vi "Dresden R2R Sputter 03.02.2018 IY24.vi"() -> ()   [LabVIEW 2009] (continued)
                                }
                                }
                                }
                                frame #1 {
                                n15635 = local read "Semi"() -> (w27616)
                                n15636 = case shown="False" w27616 {
                                frame #0 {
                                n15637 = local write "Ch1_PV18"(T/1 ("P03")) -> ()
                                n15638 = Wait Until Next ms Multiple(millisecond multiple=i32? 1000) -> ()  [unwired: 1 out]
                                }
                                frame #1 {
                                }
                                }
                                }
                                }
                              }
                              frame #1 {
                              }
                            }
                          }
                          frame #13 {
                            # "START TP"
                            n15639 = local read "Semi"() -> (w27619)
                            n15640 = case shown="False" w27619 {
                              frame #0 {
                                n15641 = stacked-sequence {
                                frame #0 {
                                n15642 = local read "Semi"() -> (w27620)
                                n15643 = case shown="False" w27620 {
                                frame #0 {
                                n15644 = stacked-sequence {
                                frame #0 {
                                n15645 = local read "Semi"() -> (w27621)
                                n15646 = case shown="False" w27621 {
                                frame #0 {
                                n15647 = local write "Tp1_auto_start"(T/1 ("Tp1_auto_start")) -> ()
                                }
                                frame #1 {
                                }
                                }
                                }
                                frame #1 {
                                n15648 = local read "Semi"() -> (w27623)
                                n15649 = case shown="False" w27623 {
                                frame #0 {
                                n15650 = Wait (ms)(milliseconds to wait=i32? 1000) -> ()  [unwired: 1 out]
                                }
                                frame #1 {
                                }
                                }
                                }
                                frame #2 {
                                n15651 = local read "Semi"() -> (w27625)
                                n15652 = case shown="False" w27625 {
                                frame #0 {
                                n15653 = while {
                                i -> [w27631]
                                stop <- w27627 stop-if-true
                                n15654 = local read "TP1_working"() -> (w27629)
                                n15655 = Greater?(x=w27631, y=i32? 120) -> (0:w27630)
                                n15656 = local read "Semi"() -> (w27628)
                                n15657 = Compound Arithmetic op=OR(w27628, w27629, w27630) -> (w27627)
                                n15658 = Wait (ms)(milliseconds to wait=i32? 500) -> ()  [unwired: 1 out]
                                }
                                }
                                frame #1 {
                                }
                                }
                                }
                                frame #3 {
                                n15659 = local read "Semi"() -> (w27633)
                                n15660 = case shown="False" w27633 {
                                frame #0 {
                                n15661 = local read "TP1_working"() -> (w27634)
                                n15662 = case shown="False" w27634 {
                                frame #0 {
                                n15663 = local write "Tp1_auto_start"(T/1 ("Pc_bv1_auto_open")) -> ()
                                }
                                frame #1 {
                                }
                                }
                                }
                                frame #1 {
                                }
                                }
                                }
                                frame #4 {
                                n15664 = local read "Semi"() -> (w27636)
                                n15665 = case shown="False" w27636 {
                                frame #0 {
                                n15666 = local read "TP1_working"() -> (w27637)
                                n15667 = case shown="False" w27637 {
                                frame #0 {
                                n15668 = Wait (ms)(milliseconds to wait=i32? 1000) -> ()  [unwired: 1 out]
                                }
                                frame #1 {
                                }
                                }
                                }
                                frame #1 {
                                }
                                }
                                }
                                frame #5 {
                                n15669 = local read "Semi"() -> (w27639)
                                n15670 = case shown="False" w27639 {
                                frame #0 {
                                n15671 = while {
                                i -> [w27645]
                                stop <- w27641 stop-if-true
                                n15672 = local read "TP1_working"() -> (w27643)
                                n15673 = Greater?(x=w27645, y=i32? 120) -> (0:w27644)
                                n15674 = local read "Semi"() -> (w27642)
                                n15675 = Compound Arithmetic op=OR(w27642, w27643, w27644) -> (w27641)
                                n15676 = Wait (ms)(milliseconds to wait=i32? 500) -> ()  [unwired: 1 out]
                                }
                                }
                                frame #1 {
                                }
                                }
                                }
                                frame #6 {
                                n15677 = local read "Semi"() -> (w27647)
                                n15678 = case shown="False" w27647 {
                                frame #0 {
                                n15679 = local read "TP1_working"() -> (w27648)
                                n15680 = case shown="False" w27648 {
                                frame #0 {
                                n15681 = local write "Error Message"("Start up process  cancelled\nbecause  TP not started.\nPlease check TP1 connections." ("Error Message")) -> ()
                                n15682 = Wait (ms)(milliseconds to wait=i32? 1000) -> ()  [unwired: 1 out]
                                }
                                frame #1 {
                                }
                                }
                                }
                                frame #1 {
                                }
                                }
                                }
                                }
                                }
                                frame #1 {
                                }
                                }
                                }
                                frame #1 {
                                n15683 = local read "Semi"() -> (w27651)
                                n15684 = case shown="False" w27651 {
                                frame #0 {
                                n15685 = local write "Ch1_PV19"(T/1 ("P03")) -> ()
                                n15686 = Wait Until Next ms Multiple(millisecond multiple=i32? 1000) -> ()  [unwired: 1 out]
                                }
                                frame #1 {
                                }
                                }
                                }
                                }
                              }
                              frame #1 {
                              }
                            }
                          }
                        }
                      }
                      frame #1 {
                      }
                    }
                  }
                  frame #1 {
                    # "PUMPING CH1 HIGHER THAN 0.9 TORR"
                    n15687 = local read "Semi"() -> (w27654)
                    n15688 = case shown="False" w27654 {
                      frame #0 {
                        n15689 = stacked-sequence {
                          frame #0 {
                            # "STOP TP"
                            n15690 = local read "Semi"() -> (w27655)
                            n15691 = case shown="False" w27655 {
                              frame #0 {
                                n15692 = stacked-sequence {
                                frame #0 {
                                n15693 = local read "Semi"() -> (w27656)
                                n15694 = case shown="False" w27656 {
                                frame #0 {
                                n15695 = stacked-sequence {
                                frame #0 {
                                n15696 = local read "Semi"() -> (w27657)
                                n15697 = case shown="False" w27657 {
                                frame #0 {
                                n15698 = local write "Tp1_auto_stop"(T/1 ("Tp1_auto_start")) -> ()
                                }
                                frame #1 {
                                }
                                }
                                }
                                frame #1 {
                                n15699 = local read "Semi"() -> (w27659)
                                n15700 = case shown="False" w27659 {
                                frame #0 {
                                n15701 = Wait (ms)(milliseconds to wait=i32? 1000) -> ()  [unwired: 1 out]
                                }
                                frame #1 {
                                }
                                }
                                }
                                frame #2 {
                                n15702 = local read "Semi"() -> (w27661)
                                n15703 = case shown="False" w27661 {
                                frame #0 {
                                n15704 = while {
                                i -> [w27667]
                                stop <- w27663 stop-if-true
                                n15705 = local read "Tp1_stopped"() -> (w27665)
                                n15706 = Greater?(x=w27667, y=i32? 120) -> (0:w27666)
                                n15707 = local read "Semi"() -> (w27664)
                                n15708 = Compound Arithmetic op=OR(w27664, w27665, w27666) -> (w27663)
                                n15709 = Wait (ms)(milliseconds to wait=i32? 500) -> ()  [unwired: 1 out]
                                }
                                }
                                frame #1 {
                                }
                                }
                                }
                                frame #3 {
                                n15710 = local read "Semi"() -> (w27669)
                                n15711 = case shown="False" w27669 {
                                frame #0 {
                                n15712 = local read "Tp1_stopped"() -> (w27670)
                                n15713 = case shown="False" w27670 {
                                frame #0 {
                                n15714 = local write "Tp1_auto_stop"(T/1 ("Pc_bv1_auto_open")) -> ()
                                }
                                frame #1 {
                                }
                                }
                                }
                                frame #1 {
                                }
                                }
                                }
                                frame #4 {
                                n15715 = local read "Semi"() -> (w27672)
                                n15716 = case shown="False" w27672 {
                                frame #0 {
                                n15717 = local read "Tp1_stopped"() -> (w27673)
                                n15718 = case shown="False" w27673 {
                                frame #0 {
                                n15719 = Wait (ms)(milliseconds to wait=i32? 1000) -> ()  [unwired: 1 out]
                                }
                                frame #1 {
                                }
                                }
                                }
                                frame #1 {
                                }
                                }
                                }
                                frame #5 {
                                n15720 = local read "Semi"() -> (w27675)
                                n15721 = case shown="False" w27675 {
                                frame #0 {
                                n15722 = while {
                                i -> [w27681]
                                stop <- w27677 stop-if-true
                                n15723 = local read "Tp1_stopped"() -> (w27679)
                                n15724 = Greater?(x=w27681, y=i32? 120) -> (0:w27680)
                                n15725 = local read "Semi"() -> (w27678)
                                n15726 = Compound Arithmetic op=OR(w27678, w27679, w27680) -> (w27677)
                                n15727 = Wait (ms)(milliseconds to wait=i32? 500) -> ()  [unwired: 1 out]
                                }
                                }
                                frame #1 {
                                }
                                }
                                }
                                frame #6 {
                                n15728 = local read "Semi"() -> (w27683)
                                n15729 = case shown="False" w27683 {
                                frame #0 {
                                n15730 = local read "Tp1_stopped"() -> (w27684)
                                n15731 = case shown="False" w27684 {
                                frame #0 {
                                n15732 = local write "Error Message"("Start up process  cancelled\nbecause  TP not stopped.\nPlease check TP1 connections." ("Error Message")) -> ()
                                n15733 = Wait (ms)(milliseconds to wait=i32? 1000) -> ()  [unwired: 1 out]
                                }
                                frame #1 {
                                }
                                }
                                }
                                frame #1 {
                                }
                                }
                                }
                                }
                                }
                                frame #1 {
                                }
                                }
                                }
                                frame #1 {
                                n15734 = local read "Semi"() -> (w27687)
                                n15735 = case shown="False" w27687 {
                                frame #0 {
                                n15736 = local write "Ch1_PA6"(T/1 ("PA2")) -> ()
                                n15737 = Wait Until Next ms Multiple(millisecond multiple=i32? 1000) -> ()  [unwired: 1 out]
                                }
                                frame #1 {
                                }
                                }
                                }
                                }
                              }
                              frame #1 {
                              }
                            }
                          }
                          frame #1 {
                            # "CLOSE CH1-CC"
                            n15738 = local read "Semi"() -> (w27690)
                            n15739 = case shown="False" w27690 {
                              frame #0 {
                                n15740 = stacked-sequence {
                                frame #0 {
                                n15741 = local read "Semi"() -> (w27691)
                                n15742 = case shown="False" w27691 {
                                frame #0 {
                                n15743 = while {
                                i -> [w27698]
                                stop <- w27692 stop-if-true
                                n15744 = Greater?(x=w27698, y=i32? 50) -> (0:w27696)
                                n15745 = case shown="True" w27696 {
                                frame #0 {
                                }
                                frame #1 {
                                n15746 = local write "Semi"(T/1 ("Semi")) -> ()
                                n15747 = local write "Error Message"("Start up process  cancelled\nbecause  CH1-CC not closed.\nPlease check  CH1-CC connections." ("Error Message")) -> ()
                                }
                                }
                                n15748 = local read "Ch1_Cc_on_off_di"() -> (w27695)
                                n15749 = case shown="True" w27695 {
                                tunnel: [T/1 i16? 0] -> w27694
                                frame #0 {
                                }
                                frame #1 {
                                n15750 = Wait Until Next ms Multiple(millisecond multiple=i32? 200) -> ()  [unwired: 1 out]
                                n15751 = local write "Ch1_Cc_on_off_do"(i16? 0 ("Ch1_Tp_bv_do")) -> ()
                                }
                                }
                                n15752 = local read "Semi"() -> (w27693)
                                n15753 = Or(x=w27694, y=w27693) -> (x .or. y?=w27692)
                                }
                                }
                                frame #1 {
                                }
                                }
                                }
                                frame #1 {
                                n15754 = local read "Semi"() -> (w27705)
                                n15755 = case shown="False" w27705 {
                                frame #0 {
                                n15756 = local write "Ch1_PA7"(T/1 ("PA3")) -> ()
                                n15757 = Wait Until Next ms Multiple(millisecond multiple=i32? 1000) -> ()  [unwired: 1 out]
                                }
                                frame #1 {
                                }
                                }
                                }
                                }
                              }
                              frame #1 {
                              }
                            }
                          }
                          frame #2 {
                            # "CLOSE BG-BV"
                            n15758 = local read "Semi"() -> (w27708)
                            n15759 = case shown="False" w27708 {
                              frame #0 {
                                n15760 = stacked-sequence {
                                frame #0 {
                                n15761 = local read "Semi"() -> (w27709)
                                n15762 = case shown="False" w27709 {
                                frame #0 {
                                n15763 = while {
                                i -> [w27716]
                                stop <- w27710 stop-if-true
                                n15764 = Greater?(x=w27716, y=i32? 50) -> (0:w27714)
                                n15765 = case shown="True" w27714 {
                                frame #0 {
                                }
                                frame #1 {
                                n15766 = local write "Semi"(T/1 ("Semi")) -> ()
                                n15767 = local write "Error Message"("Start up process  cancelled\nbecause  BG-BV not closed.\nPlease check  BG-BV1 connections." ("Error Message")) -> ()
                                }
                                }
                                n15768 = local read "Ch1_Bg_bv_di"() -> (w27713)
                                n15769 = case shown="True" w27713 {
                                tunnel: [T/1 i16? 0] -> w27712
                                frame #0 {
                                }
                                frame #1 {
                                n15770 = Wait Until Next ms Multiple(millisecond multiple=i32? 200) -> ()  [unwired: 1 out]
                                n15771 = local write "Ch1_Bg_bv_do"(i16? 0 ("Ch1_Tp_bv_do")) -> ()
                                }
                                }
                                n15772 = local read "Semi"() -> (w27711)
                                n15773 = Or(x=w27712, y=w27711) -> (x .or. y?=w27710)
                                }
                                }
                                frame #1 {
                                }
                                }
                                }
                                frame #1 {
                                n15774 = local read "Semi"() -> (w27723)
                                n15775 = case shown="False" w27723 {
                                frame #0 {
                                n15776 = local write "Ch1_PA8"(T/1 ("PA3")) -> ()
                                n15777 = Wait Until Next ms Multiple(millisecond multiple=i32? 1000) -> ()  [unwired: 1 out]
                                }
                                frame #1 {
                                }
                                }
                                }
                                }
                              }
                              frame #1 {
                              }
                            }
                          }
                          frame #3 {
                            # "CLOSE TP-BV"
                            n15778 = local read "Semi"() -> (w27726)
                            n15779 = case shown="False" w27726 {
                              frame #0 {
                                n15780 = stacked-sequence {
                                frame #0 {
                                n15781 = local read "Semi"() -> (w27727)
                                n15782 = case shown="False" w27727 {
                                frame #0 {
                                n15783 = while {
                                i -> [w27734]
                                stop <- w27728 stop-if-true
                                n15784 = Greater?(x=w27734, y=i32? 50) -> (0:w27732)
                                n15785 = case shown="True" w27732 {
                                frame #0 {
                                }
                                frame #1 {
                                n15786 = local write "Semi"(T/1 ("Semi")) -> ()
                                n15787 = local write "Error Message"("Start up process  cancelled\nbecause  TP-BV not closed.\nPlease check  TP1-BV connections." ("Error Message")) -> ()
                                }
                                }
                                n15788 = local read "Ch1_Tp_bv_di"() -> (w27731)
                                n15789 = case shown="True" w27731 {
                                tunnel: [T/1 i16? 0] -> w27730
                                frame #0 {
                                }
                                frame #1 {
                                n15790 = Wait Until Next ms Multiple(millisecond multiple=i32? 200) -> ()  [unwired: 1 out]
                                n15791 = local write "Ch1_Tp_bv_do"(i16? 0 ("Ch1_Tp_bv_do")) -> ()
                                }
                                }
                                n15792 = local read "Semi"() -> (w27729)
                                n15793 = Or(x=w27730, y=w27729) -> (x .or. y?=w27728)
                                }
                                }
                                frame #1 {
                                }
                                }
                                }
                                frame #1 {
                                n15794 = local read "Semi"() -> (w27741)
                                n15795 = case shown="False" w27741 {
                                frame #0 {
                                n15796 = local write "Ch1_PA9"(T/1 ("PA5")) -> ()
                                n15797 = Wait Until Next ms Multiple(millisecond multiple=i32? 1000) -> ()  [unwired: 1 out]
                                }
                                frame #1 {
                                }
                                }
                                }
                                }
                              }
                              frame #1 {
                              }
                            }
                          }
                          frame #4 {
                            # "False PL1-ATM"
                            n15798 = local read "Semi"() -> (w27744)
                            n15799 = case shown="False" w27744 {
                              frame #0 {
                                n15800 = stacked-sequence {
                                frame #0 {
                                n15801 = local read "Semi"() -> (w27745)
                                n15802 = case shown="False" w27745 {
                                frame #0 {
                                n15803 = local write "Ch1_Pl_atm_do"(i16? 0 ("Ch1_Pl_atm_do")) -> ()
                                }
                                frame #1 {
                                }
                                }
                                }
                                frame #1 {
                                n15804 = local read "Semi"() -> (w27747)
                                n15805 = case shown="False" w27747 {
                                frame #0 {
                                n15806 = local write "Ch1_PA10"(T/1 ("PA3")) -> ()
                                n15807 = Wait Until Next ms Multiple(millisecond multiple=i32? 1000) -> ()  [unwired: 1 out]
                                }
                                frame #1 {
                                }
                                }
                                }
                                }
                              }
                              frame #1 {
                              }
                            }
                          }
                          frame #5 {
                            # "STOP MP"
                            n15808 = local read "Semi"() -> (w27750)
                            n15809 = case shown="False" w27750 {
                              frame #0 {
                                n15810 = stacked-sequence {
                                frame #0 {
                                n15811 = local read "Semi"() -> (w27751)
                                n15812 = case shown="False" w27751 {
                                frame #0 {
                                n15813 = while {
                                i -> [w27758]
                                stop <- w27752 stop-if-true
                                n15814 = Greater?(x=w27758, y=i32? 50) -> (0:w27756)
                                n15815 = case shown="True" w27756 {
                                frame #0 {
                                }
                                frame #1 {
                                n15816 = local write "Semi"(T/1 ("Semi")) -> ()
                                n15817 = local write "Error Message"("Start up process  cancelled\nbecause MP1 not stopped.\nPlease check MP1 connections." ("Error Message")) -> ()
                                }
                                }
                                n15818 = local read "Ch1_Mp_di"() -> (w27755)
                                n15819 = case shown="True" w27755 {
                                tunnel: [T/1 i16? 0] -> w27754
                                frame #0 {
                                }
                                frame #1 {
                                n15820 = Wait Until Next ms Multiple(millisecond multiple=i32? 200) -> ()  [unwired: 1 out]
                                n15821 = local write "Ch1_Mp_do"(i16? 0 ("Ch1_Tp_bv_do")) -> ()
                                }
                                }
                                n15822 = local read "Semi"() -> (w27753)
                                n15823 = Or(x=w27754, y=w27753) -> (x .or. y?=w27752)
                                }
                                }
                                frame #1 {
                                }
                                }
                                }
                                frame #1 {
                                n15824 = local read "Semi"() -> (w27765)
                                n15825 = case shown="False" w27765 {
                                frame #0 {
                                n15826 = local write "Ch1_PA11"(T/1 ("PA3")) -> ()
                                n15827 = Wait Until Next ms Multiple(millisecond multiple=i32? 1000) -> ()  [unwired: 1 out]
                                }
                                frame #1 {
                                }
                                }
                                }
                                }
                              }
                              frame #1 {
                              }
                            }
                          }
                          frame #6 {
                            # "OPEN PL-VBV1"
                            n15828 = local read "Semi"() -> (w27768)
                            n15829 = case shown="False" w27768 {
                              frame #0 {
                                n15830 = stacked-sequence {
                                frame #0 {
                                n15831 = local read "Semi"() -> (w27769)
                                n15832 = case shown="False" w27769 {
                                frame #0 {
                                n15833 = while {
                                i -> [w27776]
                                stop <- w27771 stop-if-true
                                n15834 = Greater?(x=w27776, y=i32? 50) -> (0:w27774)
                                n15835 = case shown="True" w27774 {
                                frame #0 {
                                }
                                frame #1 {
                                n15836 = local write "Semi"(T/1 ("Semi")) -> ()
                                n15837 = local write "Error Message"("Start up process  cancelled\nbecause  PL-VBV not opened.\nPlease check PL-VBV1 connections." ("Error Message")) -> ()
                                }
                                }
                                n15838 = local read "Ch1_Pl_atm_di"() -> (w27770)
                                n15839 = case shown="False" w27770 {
                                tunnel: [w27778 T/1] -> w27773
                                frame #0 {
                                n15840 = local read "Ch1_Pl_vbv_di"() -> (w27777)
                                n15841 = case shown="False" w27777 {
                                tunnel: [i16? 0 T/1] -> w27778
                                frame #0 {
                                n15842 = local write "Ch1_Pl_vbv_do"(T/1 ("Ch1_Tp_bv_do")) -> ()
                                n15843 = Wait Until Next ms Multiple(millisecond multiple=i32? 200) -> ()  [unwired: 1 out]
                                }
                                frame #1 {
                                }
                                }
                                }
                                frame #1 {
                                }
                                }
                                n15844 = local read "Semi"() -> (w27772)
                                n15845 = Or(x=w27773, y=w27772) -> (x .or. y?=w27771)
                                }
                                }
                                frame #1 {
                                }
                                }
                                }
                                frame #1 {
                                n15846 = local read "Semi"() -> (w27786)
                                n15847 = case shown="False" w27786 {
                                frame #0 {
                                n15848 = local write "Ch1_PA12"(T/1 ("PA3")) -> ()
                                n15849 = Wait Until Next ms Multiple(millisecond multiple=i32? 1000) -> ()  [unwired: 1 out]
                                }
                                frame #1 {
                                }
                                }
                                }
                                }
                              }
                              frame #1 {
                              }
                            }
                          }
                          frame #7 {
                            # "CHECK PL-PRESSURE"
                            n15850 = local read "Semi"() -> (w27789)
                            n15851 = case shown="False" w27789 {
                              frame #0 {
                                n15852 = stacked-sequence {
                                frame #0 {
                                n15853 = local read "Semi"() -> (w27790)
                                n15854 = case shown="False" w27790 {
                                frame #0 {
                                n15855 = while {
                                i -> [w27797]
                                stop <- w27792 stop-if-true
                                n15856 = Greater?(x=w27797, y=i32? 50) -> (0:w27795)
                                n15857 = case shown="True" w27795 {
                                frame #0 {
                                }
                                frame #1 {
                                n15858 = local write "Semi"(T/1 ("Semi")) -> ()
                                n15859 = local write "Error Message"("Start up process  cancelled\nbecause  PL-ATM not opened.\nPlease check PL-ATM connections." ("Error Message")) -> ()
                                }
                                }
                                n15860 = local read "Ch1_Pl_atm_di"() -> (w27791)
                                n15861 = case shown="True" w27791 {
                                tunnel: [i16? 0 T/1] -> w27794
                                frame #0 {
                                }
                                frame #1 {
                                n15862 = Wait Until Next ms Multiple(millisecond multiple=i32? 500) -> ()  [unwired: 1 out]
                                }
                                }
                                n15863 = local read "Semi"() -> (w27793)
                                n15864 = Or(x=w27794, y=w27793) -> (x .or. y?=w27792)
                                }
                                }
                                frame #1 {
                                }
                                }
                                }
                                frame #1 {
                                n15865 = local read "Semi"() -> (w27803)
                                n15866 = case shown="False" w27803 {
                                frame #0 {
                                n15867 = local write "Ch1_PA13"(T/1 ("PA3")) -> ()
                                n15868 = Wait Until Next ms Multiple(millisecond multiple=i32? 1000) -> ()  [unwired: 1 out]
                                }
                                frame #1 {
                                }
                                }
                                }
                                }
                              }
                              frame #1 {
                              }
                            }
                          }
                          frame #8 {
                            # "False CH1-ATM"
                            n15869 = local read "Semi"() -> (w27806)
                            n15870 = case shown="False" w27806 {
                              frame #0 {
                                n15871 = stacked-sequence {
                                frame #0 {
                                n15872 = local read "Semi"() -> (w27807)
                                n15873 = case shown="False" w27807 {
                                frame #0 {
                                n15874 = local write "Ch1_Ch_atm_do"(i16? 0 ("Ch1_Pl_atm_do")) -> ()
                                }
                                frame #1 {
                                }
                                }
                                }
                                frame #1 {
                                n15875 = local read "Semi"() -> (w27809)
                                n15876 = case shown="False" w27809 {
                                frame #0 {
                                n15877 = local write "Ch1_PA14"(T/1 ("PA3")) -> ()
                                n15878 = Wait Until Next ms Multiple(millisecond multiple=i32? 1000) -> ()  [unwired: 1 out]
                                }
                                frame #1 {
                                }
                                }
                                }
                                }
                              }
                              frame #1 {
                              }
                            }
                          }
                          frame #9 {
                            # "OPEN PC-BV"
                            n15879 = local read "Semi"() -> (w27812)
                            n15880 = case shown="False" w27812 {
                              frame #0 {
                                n15881 = stacked-sequence {
                                frame #0 {
                                n15882 = local read "Semi"() -> (w27813)
                                n15883 = case shown="False" w27813 {
                                frame #0 {
                                n15884 = stacked-sequence {
                                frame #0 {
                                n15885 = local read "Semi"() -> (w27814)
                                n15886 = case shown="False" w27814 {
                                frame #0 {
                                n15887 = local write "Pc_bv1_auto_open"(T/1 ("Tp1_auto_start")) -> ()
                                }
                                frame #1 {
                                }
                                }
                                }
                                frame #1 {
                                n15888 = local read "Semi"() -> (w27816)
                                n15889 = case shown="False" w27816 {
                                frame #0 {
                                n15890 = Wait (ms)(milliseconds to wait=i32? 1000) -> ()  [unwired: 1 out]
                                }
                                frame #1 {
                                }
                                }
                                }
                                frame #2 {
                                n15891 = local read "Semi"() -> (w27818)
                                n15892 = case shown="False" w27818 {
                                frame #0 {
                                n15893 = while {
                                i -> [w27824]
                                stop <- w27820 stop-if-true
                                n15894 = local read "Pc_bv_opened_ch1"() -> (w27822)
                                n15895 = Greater?(x=w27824, y=i32? 120) -> (0:w27823)
                                n15896 = local read "Semi"() -> (w27821)
                                n15897 = Compound Arithmetic op=OR(w27821, w27822, w27823) -> (w27820)
                                n15898 = Wait (ms)(milliseconds to wait=i32? 500) -> ()  [unwired: 1 out]
                                }
                                }
                                frame #1 {
                                }
                                }
                                }
                                frame #3 {
                                n15899 = local read "Semi"() -> (w27826)
                                n15900 = case shown="False" w27826 {
                                frame #0 {
                                n15901 = local read "Pc_bv_opened_ch1"() -> (w27827)
                                n15902 = case shown="False" w27827 {
                                frame #0 {
                                n15903 = local write "Pc_bv1_auto_open"(T/1 ("Pc_bv1_auto_open")) -> ()
                                }
                                frame #1 {
                                }
                                }
                                }
                                frame #1 {
                                }
                                }
                                }
                                frame #4 {
                                n15904 = local read "Semi"() -> (w27829)
                                n15905 = case shown="False" w27829 {
                                frame #0 {
                                n15906 = local read "Pc_bv_opened_ch1"() -> (w27830)
                                n15907 = case shown="False" w27830 {
                                frame #0 {
                                n15908 = Wait (ms)(milliseconds to wait=i32? 1000) -> ()  [unwired: 1 out]
                                }
                                frame #1 {
                                }
                                }
                                }
                                frame #1 {
                                }
                                }
                                }
                                frame #5 {
                                n15909 = local read "Semi"() -> (w27832)
                                n15910 = case shown="False" w27832 {
                                frame #0 {
                                n15911 = while {
                                i -> [w27838]
                                stop <- w27834 stop-if-true
                                n15912 = local read "Pc_bv_opened_ch1"() -> (w27836)
                                n15913 = Greater?(x=w27838, y=i32? 120) -> (0:w27837)
                                n15914 = local read "Semi"() -> (w27835)
                                n15915 = Compound Arithmetic op=OR(w27835, w27836, w27837) -> (w27834)
                                n15916 = Wait (ms)(milliseconds to wait=i32? 500) -> ()  [unwired: 1 out]
                                }
                                }
                                frame #1 {
                                }
                                }
                                }
                                frame #6 {
                                n15917 = local read "Semi"() -> (w27840)
                                n15918 = case shown="False" w27840 {
                                frame #0 {
                                n15919 = local read "Pc_bv_opened_ch1"() -> (w27841)
                                n15920 = case shown="False" w27841 {
                                frame #0 {
                                n15921 = local write "Error Message"("Start up process  cancelled\nbecause  PC-BV not opened.\nPlease check PC-BV1 connections." ("Error Message")) -> ()
                                n15922 = Wait (ms)(milliseconds to wait=i32? 1000) -> ()  [unwired: 1 out]
                                }
                                frame #1 {
                                }
                                }
                                }
                                frame #1 {
                                }
                                }
                                }
                                }
                                }